vi "HFRR ADV v039.vi"() -> ()   [LabVIEW 2025] (continued)
            n794 = local write "Friction Force Tab"(T25."Page 1" ("Friction Force Tab")) -> ()
            n795 = local write "Main Calibration Tab"(T7."Main" ("Main Calibration Tab")) -> ()
          }
        }
      }
      event "FF CONTINUE": Value Change {
        n796 = event-data() -> ()  [unwired: 1 in, 6 out]
        n797 = local write "FF CONTINUE"(FALSE ("FF CONTINUE")) -> ()
        n798 = local write "Friction Force Tab"(T25."Page 2" ("Friction Force Tab")) -> ()
      }
      event "FF CONTINUE 2": Value Change {
        n799 = event-data() -> ()  [unwired: 1 in, 6 out]
        n800 = local write "FF CONTINUE 2"(FALSE ("FF CONTINUE")) -> ()
        n801 = local write "Friction Force Tab"(T25."Page 3" ("Friction Force Tab")) -> ()
      }
      event "FF CONTINUE 3": Value Change {
        n802 = event-data() -> ()  [unwired: 1 in, 6 out]
        n803 = local write "FF CONTINUE 3"(FALSE ("FF CONTINUE")) -> ()
        n804 = local write "Friction Force Tab"(T25."Page 4" ("Friction Force Tab")) -> ()
      }
      event "FF CONTINUE 4": Value Change {
        n805 = event-data() -> ()  [unwired: 1 in, 6 out]
        n806 = local write "FF CONTINUE 4"(FALSE ("FF CONTINUE")) -> ()
        n807 = local write "Friction Force Tab"(T25."Page 5" ("Friction Force Tab")) -> ()
      }
      event "FF CONTINUE 5": Value Change {
        n808 = event-data() -> ()  [unwired: 1 in, 6 out]
        n809 = local write "FF CONTINUE 5"(FALSE ("FF CONTINUE")) -> ()
        n810 = local write "Friction Force Tab"(T25."Page 6" ("Friction Force Tab")) -> ()
      }
      event "Quit": Value Change {
        n811 = event-data() -> ()  [unwired: 1 in, 6 out]
      }
    }
    n812 = Wait (ms)(milliseconds to wait=u32 100) -> ()  [unwired: 1 out]
  }
  n813 = while {
    shift-right: [w834] -> _
    shift-left: "Enum - Selector" -> [w835]
    stop <- w836 stop-if-true
    # "Auto Start Logic Loop"
    n814 = case shown="\"close\"" w835 {
      tunnel: [w839 w845 w872 w904 w934 Auto_Start_enum."Exit" ("Enum - Selector") Auto_Start_enum."Init" ("Enum - Selector")] -> w834
      frame "Init", Default {
        n815 = local read "Auto Start Test"() -> (w838:bool)
        n816 = Select(t=Auto_Start_enum."Humidity & Temperature On" ("Enum - Selector"), s=w838, f=Auto_Start_enum."Init") -> (s? t:f=w839:T15)
      }
      frame "Humidity & Temperature On" {
        n817 = stacked-sequence {
          tunnel: [_ _ _ _ _ _ Auto_Start_enum."Reach point" ("Enum - Selector")] -> w842
          frame #0 {
            w847 = T19."Disabled and Grayed Out" ("Disabled")
            w848 = TRUE ("Heater Button")
            n818 = property on="Humidity" class="Bool (strict)"("DisabledEnum"=w847) -> ()  [unwired: 2 in, 2 out]
            n819 = property on="Heater Button" class="Bool (strict)"("DisabledEnum"=w847) -> ()  [unwired: 2 in, 2 out]
            n820 = local write "Heater Button"(w848) -> ()
            n821 = local write "Humidity"(w848) -> ()
            n822 = property on="Heater Button" class="Bool (strict)"("Val(Sgnl)"=TRUE ("Value (Signaling)")) -> ()  [unwired: 2 in, 2 out]
          }
          frame #1 {
            n823 = Wait (ms)(milliseconds to wait=u32 3000) -> ()  [unwired: 1 out]
          }
          frame #2 {
            n824 = local read "Set Temp"() -> (w854:dbl)
            n825 = Number To Fractional String(number=w854, precision (6)=i16 2) -> (F-format string=w851:string)  [unwired: 2 in]
            n826 = Concatenate Strings("ST;" ("Command"), w851) -> (w852:string)
            n827 = local write "Due Write"(w852) -> ()
          }
          frame #3 {
            n828 = Wait (ms)(milliseconds to wait=u32 1500) -> ()  [unwired: 1 out]
          }
          frame #4 {
            (unwired) i16 2 ("precision (6)")
            n829 = local read "WriteHumidity"() -> (w856:string[])
            n830 = local read "Set Rh"() -> (w859:dbl)
            n831 = Number To Fractional String(number=w859) -> (F-format string=w860:string)  [unwired: 3 in]
            n832 = Concatenate Strings("M;" ("new element/subarray"), w860) -> (w861:string)
            n833 = Insert Into Array(array=w856, new element=w861) -> (w857:string[])  [unwired: 1 in]
            n834 = local write "WriteHumidity"(w857) -> ()
            n835 = local write "Due Write"("HE;1" ("Command")) -> ()
          }
          frame #5 {
            n836 = Wait (ms)(milliseconds to wait=u32 1500) -> ()  [unwired: 1 out]
          }
          frame #6 {
            w864 = TRUE ("Reach point temp")
            n837 = local write "Reach point Humidity"(w864) -> ()
            n838 = local write "Reach point temp"(w864) -> ()
          }
        }
        n839 = local read "Auto Start Test"() -> (w844:bool)
        n840 = Not(x=w844) -> (.not. x?=w843:bool)
        n841 = Select(t=Auto_Start_enum."close", s=w843, f=w842) -> (s? t:f=w845:T15)
      }
      frame "Reach point" {
        w873 = TRUE ("PAUSE")
        w881 = 1.0 ("y")
        w884 = 1.0 ("y")
        n842 = local read "Set Temp"() -> (w866:dbl)
        n843 = local read "Set Humidity:"() -> (w880:dbl)
        n844 = local read "Humidity ( %RH )"() -> (w885:dbl)
        n845 = Add(x=w866, y=w884) -> (x+y=w883:dbl)
        n846 = Subtract(x=w866, y=w884) -> (x-y=w882:dbl)
        n847 = Add(x=w880, y=w881) -> (x+y=w879:dbl)
        n848 = Subtract(x=w880, y=w881) -> (x-y=w878:dbl)
        n849 = local read "TEMP"() -> (w886:dbl)
        n850 = In Range and Coerce(upper limit=w879, x=w885, lower limit=w878) -> (In Range?=w867:bool)  [unwired: 1 out]
        n851 = In Range and Coerce(upper limit=w883, x=w886, lower limit=w882) -> (In Range?=w868:bool)  [unwired: 1 out]
        n852 = case shown="True" w867 {
          frame False {
          }
          frame True {
            n853 = case shown="True" "Reach point Humidity" {
              selector: "Reach point Humidity" -> [_ w892]
              frame False {
              }
              frame True {
                n854 = local read "EVENT LOG"() -> (w889:string)
                n855 = Not(x=w892) -> (.not. x?=w891:bool)
                n856 = local write "Reach point Humidity"(w891) -> ()
                n857 = call "Event Log.vi"("Content"="Target Humidity reached", "EVENT LOG"=w889) -> ("EVENT LOG"=w890:string)  [unwired: 8 in, 1 out]
                n858 = local write "EVENT LOG"(w890) -> ()
              }
            }
          }
        }
        n859 = case shown="True" w868 {
          frame False {
          }
          frame True {
            n860 = case shown="True" "Reach point temp" {
              selector: "Reach point temp" -> [_ w898]
              frame False {
              }
              frame True {
                n861 = local read "EVENT LOG"() -> (w895:string)
                n862 = Not(x=w898) -> (.not. x?=w897:bool)
                n863 = local write "Reach point temp"(w897) -> ()
                n864 = call "Event Log.vi"("Content"="Target Temperature reached", "EVENT LOG"=w895) -> ("EVENT LOG"=w896:string)  [unwired: 8 in, 1 out]
                n865 = local write "EVENT LOG"(w896) -> ()
              }
            }
          }
        }
        n866 = local read "Auto Start Test"() -> (w871:bool)
        n867 = And(x=w868, y=w867) -> (x .and. y?=w877:bool)
        n868 = Select(t=Auto_Start_enum."Maintain Stage" ("Enum - Selector"), s=w877, f=Auto_Start_enum."Reach point" ("Enum - Selector")) -> (s? t:f=w874:T15)
        n869 = Not(x=w871) -> (.not. x?=w870:bool)
        n870 = Select(t=Auto_Start_enum."close", s=w870, f=w874) -> (s? t:f=w872:T15)
        n871 = call "ELAPSED TIMER VI.vi"("RESET"=w873, "PAUSE"=w873) -> ()  [unwired: 7 in, 3 out]
      }
      frame "Maintain Stage" {
        w913 = 2.0 ("y")
        w912 = 1.0 ("y")
        # "Humidity and  temperatures Set Point  have been reached"
        n872 = local read "Set Temp"() -> (w899:dbl)
        n873 = local read "Set Humidity:"() -> (w916:dbl)
        n874 = local read "Humidity ( %RH )"() -> (w919:dbl)
        n875 = Add(x=w899, y=w912) -> (x+y=w918:dbl)
        n876 = Subtract(x=w899, y=w912) -> (x-y=w917:dbl)
        n877 = local read "TEMP"() -> (w920:dbl)
        n878 = Add(x=w916, y=w913) -> (x+y=w915:dbl)
        n879 = Subtract(x=w916, y=w913) -> (x-y=w914:dbl)
        n880 = In Range and Coerce(upper limit=w918, x=w920, lower limit=w917) -> (In Range?=w911:bool)  [unwired: 1 out]
        n881 = In Range and Coerce(upper limit=w915, x=w919, lower limit=w914) -> (In Range?=w910:bool)  [unwired: 1 out]
        n882 = And(x=w911, y=w910) -> (x .and. y?=w909:bool)
        n883 = Not(x=w909) -> (.not. x?=w908:bool)
        n884 = call "ELAPSED TIMER VI.vi"("TARGET"=60.0, "RESET"=w908, "PAUSE"=FALSE) -> ("ELAPSED INDICATION"=w905:bool)  [unwired: 6 in, 2 out]
        n885 = case shown="True" w905 {
          tunnel: w905 -> [_ w923]
          tunnel: [Auto_Start_enum."Maintain Stage" ("Enum - Selector") w922] -> w903
          frame False {
          }
          frame True {
            n886 = stacked-sequence {
              tunnel: w923 -> [_ _ _ _ _]
              tunnel: [_ _ _ _ Auto_Start_enum."Start Stage" ("Enum - Selector")] -> w922
              frame #0 {
                n887 = local read "EVENT LOG"() -> (w925:string)
                n888 = call "Event Log.vi"("Content"="Humidity and temperature set point has stabilized.", "EVENT LOG"=w925) -> ("EVENT LOG"=w926:string)  [unwired: 8 in, 1 out]
                n889 = local write "EVENT LOG"(w926) -> ()
              }
              frame #1 {
                n890 = Wait (ms)(milliseconds to wait=u32 100) -> ()  [unwired: 1 out]
              }
              frame #2 {
                n891 = local read "EVENT LOG"() -> (w929:string)
                n892 = call "Event Log.vi"("Content"="Auto Test Started", "EVENT LOG"=w929) -> ("EVENT LOG"=w930:string)  [unwired: 8 in, 1 out]
                n893 = local write "EVENT LOG"(w930) -> ()
              }
              frame #3 {
                w931 = TRUE ("RUN")
                n894 = local write "RUN"(w931) -> ()
                n895 = property on="Auto Start Temp" class="Bool (strict)"("Val(Sgnl)"=w931) -> ()  [unwired: 2 in, 2 out]
                "Auto Start Temp" <- w931
              }
              frame #4 {
              }
            }
          }
        }
        n896 = local read "Auto Start Test"() -> (w902:bool)
        n897 = Not(x=w902) -> (.not. x?=w901:bool)
        n898 = Select(t=Auto_Start_enum."close", s=w901, f=w903) -> (s? t:f=w904:T15)
      }
      frame "Start Stage" {
        w933 = TRUE ("PAUSE")
        n899 = local read "Auto Start Test"() -> (w938:bool)
        n900 = Not(x=w938) -> (.not. x?=w937:bool)
        n901 = Select(t=Auto_Start_enum."close" ("Enum - Selector"), s=w937, f=Auto_Start_enum."Start Stage" ("Enum - Selector")) -> (s? t:f=w934:T15)
        n902 = call "ELAPSED TIMER VI.vi"("RESET"=w933, "PAUSE"=w933) -> ()  [unwired: 7 in, 3 out]
      }
      frame "close" {
        w941 = FALSE ("Heater Button")
        n903 = local write "RUN"(w941) -> ()
        n904 = local write "Heater Button"(w941) -> ()
        n905 = local write "Humidity"(w941) -> ()
        n906 = local write "Auto Start Test"(w941) -> ()
        n907 = property on="Heater Button" class="Bool (strict)"("Val(Sgnl)"=FALSE ("Value (Signaling)")) -> ()  [unwired: 2 in, 2 out]
        n908 = local write "Humidity 2"(TRUE ("Humidity")) -> ()
      }
      frame "Exit" {
      }
    }
    n909 = Wait (ms)(milliseconds to wait=u32 100) -> ()  [unwired: 1 out]
    n910 = local read "Quit"() -> (w836:bool)
  }
  n911 = property on="Service Password Log" class="Str"("Visible"=w21) -> ()  [unwired: 2 in, 2 out]
  n912 = property on="Password 3" class="Clust (strict)"("Visible"=w21) -> ()  [unwired: 2 in, 2 out]
  n913 = while {
    stop <- w970 stop-if-true
    w953 = errorcluster {"status"=FALSE, "code"=0, "source"=""} ("error in (no error) 3")
    # "this loop is for manual report generation"
    n914 = local read "Confirm Measrurement"() -> (w952:bool)
    n915 = case shown="True" w952 {
      selector: w952 -> [_ w1060]
      tunnel: errorcluster {"status"=FALSE, "code"=0, "source"=""} ("error in (no error) 3") -> [_ w1061]
      tunnel: [_ w1059] -> _
      frame False {
      }
      frame True {
        n916 = stacked-sequence {
          tunnel: w1061 -> [_ w1094 _]
          tunnel: w1060 -> [_ _ w1201]
          tunnel: [_ w1082 _] -> w1059
          frame #0 {
            n917 = String To Path(string="C:\\LAB-IQ\\Image Calibrate v01.dcf") -> (path=w1064:path)
            n918 = Open/Create/Replace File ("Open File")(file path (use dialog)=w1064) -> (refnum out=w1065:refnum<file>)  [unwired: 5 in, 2 out]
            n919 = for {
              N: 4 -> [_]
              tunnel: w1065 -> [w1071]
              i -> [w1067]
              n920 = Read from Text File ("Read File")(file (use dialog)=w1071) -> (text=w1072:string)  [unwired: 3 in, 3 out]
              n921 = String Subset(string=w1072, offset (0)=6, length (rest)=10 ("length (rest)")) -> (substring=w1068:string)
              n922 = Fract/Exp String To Number(string=w1068) -> (number=w1066:dbl)  [unwired: 3 in, 1 out]
              n923 = case shown="3" w1067 {
                tunnel: w1066 -> [w1073 w1074 _ w1075 _]
                frame 0 {
                  n924 = local write "5x Gain"(w1073) -> ()
                }
                frame 1 {
                  n925 = local write "10x Gain"(w1074) -> ()
                }
                frame 2 {
                }
                frame 3 {
                  n926 = local write "100x gain"(w1075) -> ()
                }
                frame 4, Default {
                }
              }
            }
          }
          frame #1 {
            n927 = local read "TEST STANDARD"() -> (w1077:T3)
            n928 = case shown="\"ISO 12156\"" w1077 {
              tunnel: ["ASTM D6079" "ISO 12156"] -> w1076
              frame "ASTM D6079", Default {
              }
              frame "ISO 12156" {
              }
            }
            n929 = call "IMAGE ANALYSIS.vi"("Enum"=POST_ANALYSIS_ENUM."GET MEASUREMENTS", "error in"=w1094) -> ("error out"=w1101:errorcluster)  [unwired: 8 in, 1 out]
            n930 = local read "Magnification :"() -> (w1087:string)
            n931 = call "Stall Data Flow.vim"("value in"=w1101, "milliseconds to wait"=u32 1000) -> ("value out"=w1100:errorcluster)  [unwired: 1 out]
            n932 = local read "Test File List :"() -> (w1098:string)
            n933 = case shown="\"10x\"" w1087 {
              tunnel: [w1137 w1138] -> w1085
              frame "5x", Default {
                n934 = local read "5x Gain"() -> (w1137:dbl)
              }
              frame "10x" {
                # "5x"
                n935 = local read "10x Gain"() -> (w1138:dbl)
              }
            }
            n936 = call "IMAGE ANALYSIS.vi"("Enum"=POST_ANALYSIS_ENUM."READ", "error in"=w1100) -> ("error out"=w1097:errorcluster, "data out"=w1088:string)  [unwired: 8 in]
            n937 = Match Pattern(string=w1088, regular expression="\"type\": ") -> (after substring=w1092:string)  [unwired: 1 in, 3 out]
            n938 = call "IMAGE PATH CREATION PY.vi"("error in (no error)"=w1097, "File Name :"=w1098) -> ("error out"=w1096:errorcluster, "File Path"=w1084:path, "File Path String:"=w1079:string)  [unwired: 7 in]
            n939 = Match Pattern(string=w1092, regular expression=",") -> (before substring=w1078:string)  [unwired: 1 in, 3 out]
            n940 = local read "Calibration Tab"() -> (w1081:enum32{"Measrument", "Calibrate"})
            n941 = call "Stall Data Flow.vim"("value in"=w1096, "milliseconds to wait"=u32 250) -> ("value out"=w1080:errorcluster)  [unwired: 1 out]
            n942 = Equal?(x=w1078, y="\"rectangle\"") -> (x = y?=w1089:bool)
            n943 = case shown="False" w1089 {
              tunnel: w1088 -> [w1143 w1198]
              tunnel: w1085 -> [_ w1189]
              tunnel: cluster{"major":dbl, "minor":dbl, "average":dbl} {"major"=0.0, "minor"=0.0, "average"=0.0} -> [w1141 w1185]
              tunnel: [w1140 w1182] -> w1083
              tunnel: w1078 -> [w1142 _]
              tunnel: w1085 -> [w1139 _]
              frame False {
                n944 = Equal?(x=w1142, y="\"line\"") -> (x = y?=w1144:bool)
                n945 = case shown="True" w1144 {
                  tunnel: w1143 -> [_ w1159]
                  tunnel: w1141 -> [w1146 w1158]
                  tunnel: [w1146 w1156] -> w1140
                  tunnel: w1139 -> [_ w1155]
                  frame False {
                  }
                  frame True {
                    w1154 = 0.0 ("Major Axis")
                    n946 = Match Pattern(string=w1159, regular expression="\"length_px\":") -> (after substring=w1157:string)  [unwired: 1 in, 3 out]
                    n947 = property on="Major Axis" class="DigNum (strict)"("Caption.Text"="") -> ()  [unwired: 2 in, 2 out]
                    n948 = property on="Minor Axis" class="DigNum (strict)"("Caption.Text"="") -> ()  [unwired: 2 in, 2 out]
                    n949 = property on="Average" class="DigNum (strict)"("Caption.Text"="Line") -> ()  [unwired: 2 in, 2 out]
                    n950 = Fract/Exp String To Number(string=w1157, default (0 dbl)=0.0 ("default (0 DBL)")) -> (number=w1153:dbl)  [unwired: 2 in, 1 out]
                    "Pixel Value" <- w1153
                    n951 = Multiply(x=w1153, y=w1155) -> (x*y=w1166:dbl)
                    n952 = Multiply(x=w1166, y=1000.0) -> (x*y=w1149:dbl)
                    n953 = Divide(x=w1149, y=1000.0) -> (x/y=w1152:dbl)
                    n954 = local write "Measurment (mm)"(w1152) -> ()
                    n955 = Bundle By Name(cluster=w1158, "average"=w1149) -> (w1156:cluster{"major":dbl, "minor":dbl, "average":dbl})
                    n956 = Number To Fractional String(number=w1149, precision (6)=i16 1) -> (F-format string=w1148:string)  [unwired: 2 in]
                    n957 = local write "Minor Axis"(w1154) -> ()
                    n958 = local write "Major Axis"(w1154) -> ()
                    n959 = Fract/Exp String To Number(string=w1148) -> (number=w1147:dbl)  [unwired: 3 in, 1 out]
                    n960 = local write "Average"(w1147) -> ()
                  }
                }
              }
              frame True {
                w1186 = 1000.0 ("y")
                w1192 = 0.0 ("default (0 DBL)")
                n961 = Match Pattern(string=w1198, regular expression=" \"width_px\":") -> (after substring=w1196:string)  [unwired: 1 in, 3 out]
                n962 = Match Pattern(string=w1196, regular expression="\"height_px\":") -> (before substring=w1194:string, after substring=w1193:string)  [unwired: 1 in, 2 out]
                n963 = Fract/Exp String To Number(string=w1194, default (0 dbl)=w1192) -> (number=w1191:dbl)  [unwired: 2 in, 1 out]
                n964 = Fract/Exp String To Number(string=w1193, default (0 dbl)=w1192) -> (number=w1190:dbl)  [unwired: 2 in, 1 out]
                n965 = Multiply(x=w1191, y=w1189) -> (x*y=w1188:dbl)
                n966 = Multiply(x=w1190, y=w1189) -> (x*y=w1187:dbl)
                n967 = Multiply(x=w1188, y=w1186) -> (x*y=w1172:dbl)
                n968 = Multiply(x=w1187, y=w1186) -> (x*y=w1170:dbl)
                n969 = Add(x=w1172, y=w1170) -> (x+y=w1184:dbl)
                n970 = property on="Major Axis" class="DigNum (strict)"("Caption.Text"="Major Axis") -> ()  [unwired: 2 in, 2 out]
                n971 = property on="Minor Axis" class="DigNum (strict)"("Caption.Text"="Minor Axis") -> ()  [unwired: 2 in, 2 out]
                n972 = property on="Average" class="DigNum (strict)"("Caption.Text"="Average") -> ()  [unwired: 2 in, 2 out]
                n973 = Divide(x=w1184, y=2.0) -> (x/y=w1168:dbl)
                n974 = Bundle By Name(cluster=w1185, "major"=w1172, "minor"=w1170, "average"=w1168) -> (w1182:cluster{"major":dbl, "minor":dbl, "average":dbl})
                n975 = Number To Fractional String(number=w1170, precision (6)=i16 1) -> (F-format string=w1177:string)  [unwired: 2 in]
                n976 = Number To Fractional String(number=w1168, precision (6)=i16 1) -> (F-format string=w1178:string)  [unwired: 2 in]
                n977 = Number To Fractional String(number=w1172, precision (6)=i16 1) -> (F-format string=w1176:string)  [unwired: 2 in]
                n978 = Fract/Exp String To Number(string=w1177) -> (number=w1169:dbl)  [unwired: 3 in, 1 out]
                n979 = Fract/Exp String To Number(string=w1178) -> (number=w1167:dbl)  [unwired: 3 in, 1 out]
                n980 = Fract/Exp String To Number(string=w1176) -> (number=w1171:dbl)  [unwired: 3 in, 1 out]
                n981 = local write "Major Axis"(w1171) -> ()
                n982 = local write "Average"(w1167) -> ()
                n983 = local write "Minor Axis"(w1169) -> ()
              }
            }
            n984 = case shown="\"Measrument\", Default" w1081 {
              tunnel: w1084 -> [w1111 _]
              tunnel: w1083 -> [w1110 _]
              tunnel: [w1107 w1136] -> w1082
              tunnel: w1080 -> [w1109 w1136]
              tunnel: w1079 -> [w1108 _]
              tunnel: w1076 -> [w1106 _]
              frame "Measrument", Default {
                n985 = stacked-sequence {
                  tunnel: w1111 -> [w1129 _]
                  tunnel: w1110 -> [w1127 _]
                  tunnel: w1109 -> [w1125 _]
                  tunnel: w1108 -> [w1124 _]
                  tunnel: [w1119 _] -> w1107
                  tunnel: w1106 -> [w1112 _]
                  frame #0 {
                    n986 = call "IMAGE ANALYSIS.vi"("Enum"=POST_ANALYSIS_ENUM."SAVE IMAGE", "error in"=w1125, "IMAGE FILE PATH"=w1124) -> ("error out"=w1123:errorcluster)  [unwired: 7 in, 1 out]
                    n987 = call "Stall Data Flow.vim"("value in"=w1123, "milliseconds to wait"=u32 1000) -> ("value out"=w1114:errorcluster)  [unwired: 1 out]
                    n988 = local read "Test File List :"() -> (w1131:string)
                    n989 = call "IMAGE ANALYSIS.vi"("Enum"=POST_ANALYSIS_ENUM."MINIMIZE UI", "error in"=w1114) -> ("error out"=w1121:errorcluster)  [unwired: 8 in, 1 out]
                    n990 = Bundle By Name(cluster=T27 {"File Name"="", "Test Method"="", "Operator"="", "Fuel Description"="", "Date and time"=""} ("Main Ref"), "Test Method"=w1112, "File Name"=w1131) -> (w1132:T27)
                    n991 = call "Stall Data Flow.vim"("value in"=w1121, "milliseconds to wait"=u32 1500) -> ("value out"=w1116:errorcluster)  [unwired: 1 out]
                    n992 = call "duf file read.vi"("error in (no error)"=w1116, "Main Ref"=w1132) -> ("error out"=w1130:errorcluster, "Main Ref 2"=w1128:T27)  [unwired: 8 in]
                    n993 = call "DETECTION REPORT for manual.vi"("error in (no error)"=w1130, "return value 3"=w1127, "Image File Path"=w1129, "Main Ref"=w1128) -> ("error out"=w1126:errorcluster)  [unwired: 7 in]
                    n994 = call <vilib>:"Clear Errors.vi"("error in (no error)"=w1126) -> ("error out"=w1117:errorcluster)  [unwired: 5 in, 1 out]
                    n995 = call "IMAGE ANALYSIS.vi"("Enum"=POST_ANALYSIS_ENUM."MINIMIZE UI", "error in"=w1117) -> ("error out"=w1119:errorcluster)  [unwired: 8 in, 1 out]
                  }
                  frame #1 {
                    n996 = local write "Main Tab"(T2."HOME" ("Main Tab")) -> ()
                    n997 = local write "Main Dashboard Buttons"(T1."Home" ("Main Dashboard Buttons")) -> ()
                  }
                }
              }
              frame "Calibrate" {
              }
            }
          }
          frame #2 {
            n998 = Not(x=w1201) -> (.not. x?=w1200:bool)
            n999 = local write "Confirm Measrurement"(w1200) -> ()
            n1000 = local read "Calibration Tab"() -> (w1199:enum32{"Measrument", "Calibrate"})
            n1001 = case shown="\"Measrument\", Default" w1199 {
              frame "Measrument", Default {
                (unwired) T21."HOME" ("Main Tab")
                n1002 = local write "Main Tab"(T2."HOME" ("Main Tab")) -> ()
              }
              frame "Calibrate" {
              }
            }
          }
        }
      }
    }
    n1003 = local read "Humidity"() -> (w944:bool)
    n1004 = local read "Save Change"() -> (w949:bool)
    n1005 = local read "Calibrate"() -> (w950:bool)
    n1006 = local read "Auto Start Test"() -> (w945:bool)
    n1007 = case shown="True" w950 {
      selector: w950 -> [_ w1057]
      frame False {
      }
      frame True {
        n1008 = Not(x=w1057) -> (.not. x?=w1056:bool)
        n1009 = local write "Calibrate"(w1056) -> ()
        n1010 = local write "Calibration Tab"(enum32{"Measrument", "Calibrate"}."Calibrate" ("Calibration Tab")) -> ()
      }
    }
    n1011 = case shown="True" w949 {
      selector: w949 -> [_ w1001]
      frame False {
      }
      frame True {
        n1012 = stacked-sequence {
          tunnel: w1001 -> [_ _ _ _ w1055]
          frame #0 {
            n1013 = call "IMAGE ANALYSIS.vi"("Enum"=POST_ANALYSIS_ENUM."HIDE UI") -> ()  [unwired: 9 in, 2 out]
          }
          frame #1 {
            n1014 = local read "100x gain"() -> (w1003:dbl)
            n1015 = local read "10x Gain"() -> (w1004:dbl)
            n1016 = local read "5x Gain"() -> (w1005:dbl)
            n1017 = Number To Fractional String(number=w1004, width (-)=i16 4, precision (6)=i16 7) -> (F-format string=w1026:string)  [unwired: 1 in]
            n1018 = Number To Fractional String(number=0.0, width (-)=i16 4, precision (6)=i16 7) -> (F-format string=w1021:string)  [unwired: 1 in]
            n1019 = Number To Fractional String(number=w1003, width (-)=i16 4, precision (6)=i16 7) -> (F-format string=w1009:string)  [unwired: 1 in]
            n1020 = Number To Fractional String(number=w1005, width (-)=i16 10 ("precision (6)"), precision (6)=i16 7) -> (F-format string=w1035:string)  [unwired: 1 in]
            n1021 = Concatenate Strings("[CH1]" ("string"), w1035, " - 5x Gain" ("string"), "\r") -> (w1025:string)
            n1022 = Concatenate Strings("[CH2]" ("string"), w1026, " - 10x Gain" ("string"), "\r") -> (w1024:string)
            n1023 = Concatenate Strings("[CH3]" ("string"), w1021, " - 20x Gain" ("string"), "\r") -> (w1015:string)
            n1024 = Concatenate Strings("[CH4]" ("string"), w1009, " - 100x Gain" ("string"), "\r") -> (w1008:string)
            n1025 = String To Path(string="C:\\LAB-IQ\\Image Calibrate v01.dcf") -> (path=w1038:path)
            n1026 = Concatenate Strings(w1025, w1024, w1015, w1008) -> (w1023:string)
            n1027 = call <vilib>:"Write Characters To File.vi"("append to file? (new file:F)"=FALSE, "character string"=w1023, "file path (dialog if empty)"=w1038) -> ()  [unwired: 2 in, 1 out]
          }
          frame #2 {
            n1028 = String To Path(string="C:\\LAB-IQ\\Image Calibrate v01.dcf") -> (path=w1041:path)
            n1029 = Open/Create/Replace File ("Open File")(file path (use dialog)=w1041) -> (refnum out=w1042:refnum<file>)  [unwired: 5 in, 2 out]
            n1030 = for {
              N: 4 -> [_]
              tunnel: w1042 -> [w1048]
              i -> [w1044]
              n1031 = Read from Text File ("Read File")(file (use dialog)=w1048) -> (text=w1049:string)  [unwired: 3 in, 3 out]
              n1032 = String Subset(string=w1049, offset (0)=6, length (rest)=10 ("length (rest)")) -> (substring=w1045:string)
              n1033 = Fract/Exp String To Number(string=w1045) -> (number=w1043:dbl)  [unwired: 3 in, 1 out]
              n1034 = case shown="3" w1044 {
                tunnel: w1043 -> [w1050 w1051 _ w1052 _]
                frame 0 {
                  n1035 = local write "5x Gain"(w1050) -> ()
                }
                frame 1 {
                  n1036 = local write "10x Gain"(w1051) -> ()
                }
                frame 2 {
                }
                frame 3 {
                  n1037 = local write "100x gain"(w1052) -> ()
                }
                frame 4, Default {
                }
              }
            }
          }
          frame #3 {
            n1038 = call "IMAGE ANALYSIS.vi"("Enum"=POST_ANALYSIS_ENUM."SHOW UI") -> ()  [unwired: 9 in, 2 out]
          }
          frame #4 {
            n1039 = Not(x=w1055) -> (.not. x?=w1054:bool)
            n1040 = local write "Save Change"(w1054) -> ()
          }
        }
      }
    }
    n1041 = case shown="False" w945 {
      tunnel: w944 -> [w971 _]
      frame False {
        n1042 = case shown="True" w971 {
          frame False {
          }
          frame True {
            n1043 = local read "Set Humidity:"() -> (w975:dbl)
            n1044 = local read "Set Humidity:"() -> (w978:dbl)
            n1045 = local read "Humidity ( %RH )"() -> (w979:dbl)
            n1046 = Subtract(x=w975, y=2.0) -> (x-y=w973:dbl)
            n1047 = Add(x=w978, y=2.0) -> (x+y=w974:dbl)
            n1048 = In Range and Coerce(upper limit=w974, x=w979, lower limit=w973) -> (In Range?=w972:bool)  [unwired: 1 out]
            n1049 = case shown="True" w972 {
              frame False {
              }
              frame True {
                n1050 = case shown="True" "Manual Humididty Reached" {
                  selector: "Manual Humididty Reached" -> [_ w982]
                  frame False {
                  }
                  frame True {
                    n1051 = Not(x=w982) -> (.not. x?=w981:bool)
                    n1052 = local write "Manual Humididty Reached"(w981) -> ()
                    n1053 = local read "EVENT LOG"() -> (w984:string)
                    n1054 = call "Event Log.vi"("Content"="Target Humidity reached", "EVENT LOG"=w984) -> ("EVENT LOG"=w983:string)  [unwired: 8 in, 1 out]
                    n1055 = local write "EVENT LOG"(w983) -> ()
                  }
                }
              }
            }
          }
        }
      }
      frame True {
        n1056 = local write "Manual Humididty Reached"(TRUE ("Manual Humididty Reached")) -> ()
      }
    }
    n1057 = local read "Cap Live Image"() -> (w965:bool)
    n1058 = local read "SCAR MEASURMENT"() -> (w968:enum32{"Auto Scar", "Manual Scar"})
    n1059 = Equal?(x=w968, y=enum32{"Auto Scar", "Manual Scar"}."Manual Scar" ("SCAR MEASURMENT")) -> (x = y?=w966:bool)
    n1060 = And(x=w966, y=w965) -> (x .and. y?=w964:bool)
    n1061 = Wait (ms)(milliseconds to wait=u32 250) -> ()  [unwired: 1 out]
    n1062 = case shown="True" w964 {
      selector: w964 -> [_ w1287]
      frame False {
      }
      frame True {
        n1063 = stacked-sequence {
          tunnel: [_ _ _ w1306 _] -> _
          tunnel: w1287 -> [_ _ _ _ w1313]
          frame #0 {
            w1288 = 0.0
            n1064 = local write "Major Axis"(w1288) -> ()
            n1065 = local write "Minor Axis"(w1288) -> ()
            n1066 = local write "Average"(w1288) -> ()
          }
          frame #1 {
            n1067 = call "CAMERA LIVE FEED FGV.vi"("Enum - Menu"=CAMERA_LIVE_FEED_ENUM."CAMERA MINIMIZE") -> ()  [unwired: 9 in, 2 out]
          }
          frame #2 {
            n1068 = local read "Magnification len live scar"() -> (w1292:string)
            n1069 = case shown="\"10x\", Default" w1292 {
              tunnel: ["_10x" "_5x"] -> w1291
              frame "10x", Default {
              }
              frame "5x" {
              }
            }
            n1070 = local read "FILE 3"() -> (w1298:string)
            n1071 = call <vilib>:"Trim Whitespace.vi"("string"="C:\\LAB-IQ\\images\\") -> ("trimmed string"=w1300:string)  [unwired: 1 in]
            n1072 = String To Path(string=w1300) -> (path=w1299:path)
            n1073 = Concatenate Strings(w1298, w1291, ".png" ("string")) -> (w1297:string)
            n1074 = Build Path(base path=w1299, name or relative path=w1297) -> (appended path=w1296:path)
            n1075 = Path To String(path=w1296) -> (string=w1295:string)
            n1076 = call "CAMERA LIVE FEED FGV.vi"("Enum - Menu"=CAMERA_LIVE_FEED_ENUM."CAMERA SAVE", "Image Path"=w1295) -> ("error out"=w1293:errorcluster)  [unwired: 8 in, 1 out]
            n1077 = case shown="No Error" w1293 {
              frame No Error {
                n1078 = One Button Dialog(message="Image saved successfully") -> ()  [unwired: 1 in, 1 out]
              }
              frame Error {
              }
            }
          }
          frame #3 {
            n1079 = call "LIST FILE NAMES.vi"() -> ("error out"=w1308:errorcluster, "filenames"=w1305:string[])  [unwired: 10 in]
            n1080 = call "IMAGE ANALYSIS.vi"("Enum"=POST_ANALYSIS_ENUM."SHOW UI", "error in"=w1308) -> ("error out"=w1306:errorcluster)  [unwired: 8 in, 1 out]
            n1081 = property on="Test File List :" class="CmbBox"("Strings[]"=w1305) -> ()  [unwired: 2 in, 2 out]
          }
          frame #4 {
            (unwired) T26."Report" ("Main Dashboard Buttons")
            (unwired) T28."Report" ("Main Dashboard Buttons")
            n1082 = Not(x=w1313) -> (.not. x?=w1312:bool)
            n1083 = local write "Zoom Factore"(0.0 ("Zoom Factore")) -> ()
            n1084 = local write "Cap Live Image"(w1312) -> ()
            n1085 = local write "Main Tab"(T2."Adv Scar Report" ("Main Tab")) -> ()
            n1086 = property on="Cap Live Image" class="Bool (strict)"("BoolText.Text"="Capture Image" ("Boolean Text.Text")) -> ()  [unwired: 2 in, 2 out]
            n1087 = local write "Main Dashboard Buttons"(T1."Report" ("Main Dashboard Buttons")) -> ()
          }
        }
      }
    }
    n1088 = local read "change Gain"() -> (w948:bool)
    n1089 = local read "Back Square"() -> (w947:bool)
    n1090 = case shown="True" w948 {
      selector: w948 -> [_ w992]
      frame False {
      }
      frame True {
        n1091 = stacked-sequence {
          tunnel: w992 -> [_ w1000]
          frame #0 {
            n1092 = local read "Actual (µm)"() -> (w996:dbl)
            n1093 = local read "Pixel Value"() -> (w995:dbl)
            n1094 = local read "Magnification :"() -> (w994:string)
            n1095 = Divide(x=w996, y=w995) -> (x/y=w993:dbl)
            n1096 = case shown="\"10x\"" w994 {
              tunnel: w993 -> [w997 w998]
              frame "10x" {
                n1097 = local write "10x Gain"(w997) -> ()
              }
              frame "5x", Default {
                n1098 = local write "5x Gain"(w998) -> ()
              }
            }
          }
          frame #1 {
            n1099 = Not(x=w1000) -> (.not. x?=w999:bool)
            n1100 = local write "change Gain"(w999) -> ()
          }
        }
      }
    }
    n1101 = case shown="True" w947 {
      selector: w947 -> [_ w990]
      frame False {
      }
      frame True {
        n1102 = Not(x=w990) -> (.not. x?=w989:bool)
        n1103 = local write "Back Square"(w989) -> ()
        n1104 = local write "Calibration Tab"(enum32{"Measrument", "Calibrate"}."Measrument" ("Calibration Tab")) -> ()
      }
    }
    n1105 = local read "Rectangle Tool"() -> (w959:bool)
    n1106 = local read "Clear ROI Tool"() -> (w958:bool)
    n1107 = local read "Open Image"() -> (w963:bool)
    n1108 = local read "line tool"() -> (w960:bool)
    n1109 = local read "OUT"() -> (w961:bool)
    n1110 = local read "In"() -> (w962:bool)
    n1111 = case shown="True" w963 {
      selector: w963 -> [_ w1273]
      tunnel: [w1264 w1275] -> _
      tunnel: w953 -> [w1264 w1274]
      frame False {
      }
      frame True {
        w1268 = "_5x" ("regular expression")
        n1112 = Not(x=w1273) -> (.not. x?=w1272:bool)
        n1113 = local write "Open Image"(w1272) -> ()
        n1114 = call "IMAGE ANALYSIS.vi"("Enum"=POST_ANALYSIS_ENUM."HIDE UI", "error in"=w1274) -> ("error out"=w1282:errorcluster)  [unwired: 8 in, 1 out]
        n1115 = call <vilib>:"Clear Errors.vi"("error in (no error)"=w1282) -> ("error out"=w1265:errorcluster)  [unwired: 5 in, 1 out]
        n1116 = call "File Dialog"("start path"=path "C:/LAB-IQ/images", "error in"=w1265) -> ("selected path"=w1267:path, "error out"=w1280:errorcluster)  [unwired: 10 in, 2 out]
        "Image path  2" <- w1267
        n1117 = call <vilib>:"Clear Errors.vi"("error in (no error)"=w1280) -> ("error out"=w1279:errorcluster)  [unwired: 5 in, 1 out]
        n1118 = call "IMAGE ANALYSIS.vi"("Enum"=POST_ANALYSIS_ENUM."OPEN FILE", "error in"=w1279, "File Path"=w1267) -> ("error out"=w1278:errorcluster)  [unwired: 7 in, 1 out]
        n1119 = call <vilib>:"Clear Errors.vi"("error in (no error)"=w1278) -> ("error out"=w1277:errorcluster)  [unwired: 5 in, 1 out]
        n1120 = call "IMAGE ANALYSIS.vi"("Enum"=POST_ANALYSIS_ENUM."SHOW UI", "error in"=w1277) -> ("error out"=w1275:errorcluster)  [unwired: 8 in, 1 out]
        n1121 = local write "Zoom Factore"(100.0 ("Zoom Factore")) -> ()
        n1122 = Strip Path(path=w1267) -> (name=w1270:string)  [unwired: 1 out]
        n1123 = Match Pattern(string=w1270, regular expression=w1268) -> (match substring=w1269:string)  [unwired: 1 in, 3 out]
        n1124 = Equal?(x=w1269, y=w1268) -> (x = y?=w1266:bool)
        n1125 = case shown="False" w1266 {
          frame False {
            n1126 = local write "Magnification :"("10x" ("Magnification :")) -> ()
          }
          frame True {
            n1127 = local write "Magnification :"("5x" ("Magnification :")) -> ()
          }
        }
      }
    }
    n1128 = case shown="True" w961 {
      selector: w961 -> [_ w1249]
      tunnel: w953 -> [w1246 w1254]
      tunnel: [w1246 w1248] -> _
      frame False {
      }
      frame True {
        n1129 = Not(x=w1249) -> (.not. x?=w1247:bool)
        n1130 = local read "Zoom Factore"() -> (w1252:dbl)
        n1131 = local write "OUT"(w1247) -> ()
        n1132 = call "IMAGE ANALYSIS.vi"("Enum"=POST_ANALYSIS_ENUM."ZOOM OUT", "error in"=w1254) -> ("error out"=w1248:errorcluster)  [unwired: 8 in, 1 out]
        n1133 = Divide(x=w1252, y=1.2) -> (x/y=w1250:dbl)
        n1134 = local write "Zoom Factore"(w1250) -> ()
      }
    }
    n1135 = case shown="True" w962 {
      selector: w962 -> [_ w1258]
      tunnel: w953 -> [w1255 w1263]
      tunnel: [w1255 w1256] -> _
      frame False {
      }
      frame True {
        n1136 = Not(x=w1258) -> (.not. x?=w1257:bool)
        n1137 = local read "Zoom Factore"() -> (w1261:dbl)
        n1138 = local write "In"(w1257) -> ()
        n1139 = call "IMAGE ANALYSIS.vi"("Enum"=POST_ANALYSIS_ENUM."ZOOM IN", "error in"=w1263) -> ("error out"=w1256:errorcluster)  [unwired: 8 in, 1 out]
        n1140 = Multiply(x=w1261, y=1.2) -> (x*y=w1259:dbl)
        n1141 = local write "Zoom Factore"(w1259) -> ()
      }
    }
    n1142 = case shown="True" w958 {
      selector: w958 -> [_ w1230]
      tunnel: w953 -> [w1228 w1232]
      tunnel: [w1228 w1231] -> _
      frame False {
      }
      frame True {
        n1143 = Not(x=w1230) -> (.not. x?=w1229:bool)
        n1144 = local write "Clear ROI Tool"(w1229) -> ()
        n1145 = call "IMAGE ANALYSIS.vi"("Enum"=POST_ANALYSIS_ENUM."CLEAR ROI", "error in"=w1232) -> ("error out"=w1231:errorcluster)  [unwired: 8 in, 1 out]
      }
    }
    n1146 = case shown="True" w960 {
      selector: w960 -> [_ w1242]
      tunnel: w953 -> [w1240 w1245]
      tunnel: [w1240 w1243] -> _
      frame False {
      }
      frame True {
        n1147 = Not(x=w1242) -> (.not. x?=w1241:bool)
        n1148 = local write "line tool"(w1241) -> ()
        n1149 = call "IMAGE ANALYSIS.vi"("Enum"=POST_ANALYSIS_ENUM."DRAW LINE", "error in"=w1245) -> ("error out"=w1243:errorcluster)  [unwired: 8 in, 1 out]
      }
    }
    n1150 = case shown="True" w959 {
      selector: w959 -> [_ w1236]
      tunnel: w953 -> [w1234 w1238]
      tunnel: [w1234 w1237] -> _
      frame False {
      }
      frame True {
        n1151 = Not(x=w1236) -> (.not. x?=w1235:bool)
        n1152 = local write "Rectangle Tool"(w1235) -> ()
        n1153 = call "IMAGE ANALYSIS.vi"("Enum"=POST_ANALYSIS_ENUM."DRAW REC", "error in"=w1238) -> ("error out"=w1237:errorcluster)  [unwired: 8 in, 1 out]
      }
    }
    n1154 = local read "SCAR MEASURMENT"() -> (w946:enum32{"Auto Scar", "Manual Scar"})
    n1155 = local read "Fit to Screen Tool"() -> (w955:bool)
    n1156 = local read "Resize Tool"() -> (w954:bool)
    n1157 = case shown="\"Manual Scar\", Default" w946 {
      frame "Auto Scar" {
        n1158 = property on="Cap Live Image" class="Bool (strict)"("BoolText.Text"="Report" ("Boolean Text.Text")) -> ()  [unwired: 2 in, 2 out]
      }
      frame "Manual Scar", Default {
        n1159 = property on="Cap Live Image" class="Bool (strict)"("BoolText.Text"="Save Image" ("Boolean Text.Text")) -> ()  [unwired: 2 in, 2 out]
      }
    }
    n1160 = local read "ROI Color Tool"() -> (w956:bool)
    n1161 = local read "Pan Tool"() -> (w957:bool)
    n1162 = case shown="True" w957 {
      selector: w957 -> [_ w1224]
      tunnel: w953 -> [w1222 w1226]
      tunnel: [w1222 w1225] -> _
      frame False {
      }
      frame True {
        n1163 = Not(x=w1224) -> (.not. x?=w1223:bool)
        n1164 = call "IMAGE ANALYSIS.vi"("Enum"=POST_ANALYSIS_ENUM."PAN", "error in"=w1226) -> ("error out"=w1225:errorcluster)  [unwired: 8 in, 1 out]
        n1165 = local write "Pan Tool"(w1223) -> ()
      }
    }
    n1166 = case shown="True" w954 {
      selector: w954 -> [_ w1208]
      tunnel: w953 -> [w1203 w1205]
      tunnel: [w1203 w1204] -> _
      frame False {
      }
      frame True {
        n1167 = Not(x=w1208) -> (.not. x?=w1207:bool)
        n1168 = local write "Resize Tool"(w1207) -> ()
        n1169 = call "IMAGE ANALYSIS.vi"("Enum"=POST_ANALYSIS_ENUM."RESIZE MODE", "error in"=w1205) -> ("error out"=w1204:errorcluster)  [unwired: 8 in, 1 out]
      }
    }
    n1170 = case shown="True" w955 {
      selector: w955 -> [_ w1213]
      tunnel: [w1209 w1214] -> _
      tunnel: w953 -> [w1209 w1212]
      frame False {
      }
      frame True {
        n1171 = Not(x=w1213) -> (.not. x?=w1211:bool)
        n1172 = local write "Zoom Factore"(100.0 ("Zoom Factore")) -> ()
        n1173 = local write "Fit to Screen Tool"(w1211) -> ()
        n1174 = call "IMAGE ANALYSIS.vi"("Enum"=POST_ANALYSIS_ENUM."FIT", "error in"=w1212) -> ("error out"=w1214:errorcluster)  [unwired: 8 in, 1 out]
      }
    }
    n1175 = case shown="True" w956 {
      selector: w956 -> [_ w1219]
      tunnel: [w1216 w1220] -> _
      tunnel: w953 -> [w1216 w1217]
      frame False {
      }
      frame True {
        n1176 = Not(x=w1219) -> (.not. x?=w1218:bool)
        n1177 = local write "ROI Color Tool"(w1218) -> ()
        n1178 = call "IMAGE ANALYSIS.vi"("Enum"=POST_ANALYSIS_ENUM."SET ROI COLOR", "error in"=w1217) -> ("error out"=w1220:errorcluster)  [unwired: 8 in, 1 out]
      }
    }
    n1179 = local read "Quit"() -> (w970:bool)
  }
  n1180 = while {
    stop <- w1315 stop-if-true
    n1181 = local read "Image Path"() -> (w1318:path)
    n1182 = local read "Print 3"() -> (w1321:bool)
    n1183 = Equal?(x=w1318, y=path "") -> (x = y?=w1317:bool)
    n1184 = Not(x=w1317) -> (.not. x?=w1316:bool)
    n1185 = property on="Print 3" class="Bool (strict)"("Visible"=w1316) -> ()  [unwired: 2 in, 2 out]
    n1186 = case shown="True" w1321 {
      frame False {
        n1187 = local write "Rd"(TRUE ("Boolean 7")) -> ()
      }
      frame True {
        n1188 = flat-sequence {
          tunnel: [w1361] -> w1329
          tunnel: [w1348] -> w1327
          tunnel: [w1358] -> w1323
          tunnel: w1329 -> [w1370]
          tunnel: [w1370] -> w1328
          tunnel: w1327 -> [w1369]
          tunnel: [w1369] -> w1326
          tunnel: [w1367] -> w1325
          tunnel: [w1366] -> w1324
          tunnel: w1323 -> [w1366]
          tunnel: w1328 -> [w1372]
          tunnel: w1326 -> [w1373]
          tunnel: w1325 -> [_]
          tunnel: w1324 -> [w1371]
          frame #0 {
            n1189 = case shown="True" "Rd" {
              frame False {
              }
              frame True {
                n1190 = while {
                  tunnel: "abcdefABCDEF" ("string 2") -> [w1340]
                  shift-right: [w1338] -> w1332
                  shift-left: "" -> [w1337]
                  i -> [w1347]
                  stop <- w1346 stop-if-true
                  n1191 = Random Number (0-1)() -> (number: 0 to 1=w1341:dbl)
                  n1192 = Multiply(x=w1341, y=62.0) -> (x*y=w1343:dbl)
                  n1193 = Decrement(x="Length 2") -> (x-1=w1336:i16)
                  n1194 = To Word Integer(number=w1343) -> (16bit integer=w1344:i16)
                  n1195 = String Subset(string=w1340, offset (0)=w1344, length (rest)=1 ("length (rest)")) -> (substring=w1339:string)
                  n1196 = Greater Or Equal?(x=w1347, y=w1336) -> (x >= y?=w1346:bool)
                  n1197 = Concatenate Strings(w1339, w1337) -> (w1338:string)
                }
                "String 10" <- w1332
                n1198 = local write "Rd"(FALSE ("Boolean 7")) -> ()
              }
            }
          }
          frame #1 {
            w1359 = "_resized.jpg" ("command line")
            (unwired) ".jpg -resize 320x240 " ("string")
            (unwired) "Choose an Image File" ("prompt")
            # "-resize 1798x425"
            n1199 = local read "Image Path"() -> (w1353:path)
            n1200 = Strip Path(path=w1353) -> (stripped path=w1348:path, name=w1349:string)
            n1201 = Match Pattern(string=w1349, regular expression=".jpg") -> (before substring=→"before substring 2":string, after substring=→"after substring":string)  [unwired: 1 in, 2 out]
            n1202 = Match Pattern(string=w1349, regular expression="\\") -> (before substring=w1355:string)  [unwired: 1 in, 3 out]
            n1203 = Match Pattern(string=w1355, regular expression=".jpg") -> (before substring=w1354:string)  [unwired: 1 in, 3 out]
            n1204 = Concatenate Strings("cmd /c convert " ("string"), w1354, ".jpg -resize 320x240  " ("command line"), w1354, w1359) -> (w1362:string)
            n1205 = call <vilib>:"System Exec.vi"("run minimized? (F)"=TRUE, "wait until completion? (T)"=TRUE, "working directory"=w1348, "command line"=w1362) -> ("error out"=w1361:errorcluster)  [unwired: 4 in, 3 out]
            "error out 2" <- w1361
            n1206 = Concatenate Strings(w1354, w1359) -> (w1358:string)
          }
          frame #2 {
            n1207 = Wait (ms)(milliseconds to wait=u32 2000 ("millisecond timer value")) -> (millisecond timer value=w1367:u32)
          }
          frame #3 {
            n1208 = case shown="No Error" w1372 {
              tunnel: w1373 -> [w1376 _]
              tunnel: w1371 -> [w1374 _]
              frame No Error {
                (unwired) ".jpg" ("string")
                n1209 = Path To String(path=w1376) -> (string=w1380:string)
                n1210 = Concatenate Strings(w1380, "\\" ("string"), w1374) -> (w1379:string)
                n1211 = String To Path(string=w1379) -> (path=w1378:path)
                n1212 = call <vilib>:"Read JPEG File.vi"("path to JPEG file"=w1378) -> ("image data"=w1382:T16)  [unwired: 8 in, 2 out]
                "image data" <- w1382
                n1213 = local write "Print 3"(FALSE ("Print 2")) -> ()
                n1214 = call <vilib>:"Draw Flattened Pixmap.vi"("image data"=w1382) -> ("new picture"=→"new picture":picture)  [unwired: 8 in]
              }
              frame Error {
              }
            }
          }
        }
      }
    }
    n1215 = Wait (ms)(milliseconds to wait=u32 20 ("millisecond timer value")) -> ()  [unwired: 1 out]
    n1216 = local read "Quit"() -> (w1315:bool)
  }
  n1217 = while {
    tunnel: w38 -> [_]
    tunnel: w24 -> [_]
    stop <- w1412 stop-if-true
    # "New Adv Logics"
    n1218 = local read "Main Tab"() -> (w1393:T2)
    n1219 = local read "Main Tab"() -> (w1410:T2)
    n1220 = local read "Sign In"() -> (w1409:bool)
    n1221 = case shown="\"Adv Scar\"" w1393 {
      frame "HOME", Default {
        n1222 = local read "LIVE FEED MIN TEMP"() -> (w1545:bool)
        n1223 = local write "LIVE FEED MAX TEMP"(TRUE ("LIVE FEED MAX TEMP")) -> ()
        n1224 = local read "CAMERA ROI MIN TEMP"() -> (w1543:bool)
        n1225 = case shown="True" w1545 {
          selector: w1545 -> [_ w1552]
          frame False {
          }
          frame True {
            n1226 = Not(x=w1552) -> (.not. x?=w1551:bool)
            n1227 = local write "LIVE FEED MIN TEMP"(w1551) -> ()
            n1228 = call "CAMERA LIVE FEED FGV.vi"("Enum - Menu"=CAMERA_LIVE_FEED_ENUM."CAMERA MINIMIZE") -> ()  [unwired: 9 in, 2 out]
          }
        }
        n1229 = case shown="True" w1543 {
          selector: w1543 -> [_ w1549]
          frame False {
          }
          frame True {
            n1230 = Not(x=w1549) -> (.not. x?=w1548:bool)
            n1231 = local write "CAMERA ROI MIN TEMP"(w1548) -> ()
            n1232 = call "IMAGE ANALYSIS.vi"("Enum"=POST_ANALYSIS_ENUM."MINIMIZE UI") -> ()  [unwired: 9 in, 2 out]
          }
        }
        n1233 = local write "CAMERA ROI MAX TEMP"(TRUE ("CAMERA ROI MAX TEMP")) -> ()
      }
      frame "Test Setup" {
        n1234 = local read "LIVE FEED MIN TEMP"() -> (w1555:bool)
        n1235 = local read "CAMERA ROI MIN TEMP"() -> (w1553:bool)
        n1236 = local write "LIVE FEED MAX TEMP"(TRUE ("LIVE FEED MAX TEMP")) -> ()
        n1237 = case shown="True" w1555 {
          selector: w1555 -> [_ w1562]
          frame False {
          }
          frame True {
            n1238 = Not(x=w1562) -> (.not. x?=w1561:bool)
            n1239 = local write "LIVE FEED MIN TEMP"(w1561) -> ()
            n1240 = call "CAMERA LIVE FEED FGV.vi"("Enum - Menu"=CAMERA_LIVE_FEED_ENUM."CAMERA MINIMIZE") -> ()  [unwired: 9 in, 2 out]
          }
        }
        n1241 = case shown="True" w1553 {
          selector: w1553 -> [_ w1559]
          frame False {
          }
          frame True {
            n1242 = Not(x=w1559) -> (.not. x?=w1558:bool)
            n1243 = local write "CAMERA ROI MIN TEMP"(w1558) -> ()
            n1244 = call "IMAGE ANALYSIS.vi"("Enum"=POST_ANALYSIS_ENUM."MINIMIZE UI") -> ()  [unwired: 9 in, 2 out]
          }
        }
        n1245 = local write "CAMERA ROI MAX TEMP"(TRUE ("CAMERA ROI MAX TEMP")) -> ()
      }
      frame "Acquire" {
        n1246 = local read "LIVE FEED MIN TEMP"() -> (w1565:bool)
        n1247 = local write "LIVE FEED MAX TEMP"(TRUE ("LIVE FEED MAX TEMP")) -> ()
        n1248 = local read "CAMERA ROI MIN TEMP"() -> (w1563:bool)
        n1249 = case shown="True" w1565 {
          selector: w1565 -> [_ w1572]
          frame False {
          }
          frame True {
            n1250 = Not(x=w1572) -> (.not. x?=w1571:bool)
            n1251 = local write "LIVE FEED MIN TEMP"(w1571) -> ()
            n1252 = call "CAMERA LIVE FEED FGV.vi"("Enum - Menu"=CAMERA_LIVE_FEED_ENUM."CAMERA MINIMIZE") -> ()  [unwired: 9 in, 2 out]
          }
        }
        n1253 = case shown="True" w1563 {
          selector: w1563 -> [_ w1569]
          frame False {
          }
          frame True {
            n1254 = Not(x=w1569) -> (.not. x?=w1568:bool)
            n1255 = local write "CAMERA ROI MIN TEMP"(w1568) -> ()
            n1256 = call "IMAGE ANALYSIS.vi"("Enum"=POST_ANALYSIS_ENUM."MINIMIZE UI") -> ()  [unwired: 9 in, 2 out]
          }
        }
        n1257 = local write "CAMERA ROI MAX TEMP"(TRUE ("CAMERA ROI MAX TEMP")) -> ()
      }
      frame "Adv Scar" {
        n1258 = local read "CAMERA ROI MIN TEMP"() -> (w1573:bool)
        n1259 = case shown="True" "LIVE FEED MAX TEMP" {
          selector: "LIVE FEED MAX TEMP" -> [_ w1594]
          frame False {
          }
          frame True {
            n1260 = Not(x=w1594) -> (.not. x?=w1593:bool)
            n1261 = local write "LIVE FEED MAX TEMP"(w1593) -> ()
            n1262 = call "CAMERA LIVE FEED FGV.vi"("Enum - Menu"=CAMERA_LIVE_FEED_ENUM."CAMERA RESTORE") -> ("error out"=w1584:errorcluster)  [unwired: 9 in, 1 out]
            n1263 = Type Cast(type=30, x=0) -> (*(type *) &x=w1588:i32)
            n1264 = Add(x=w1588, y=48) -> (x+y=w1589:i32)
            n1265 = call "CAMERA LIVE FEED FGV.vi"("Enum - Menu"=CAMERA_LIVE_FEED_ENUM."CAMERA MODE SET", "error in (no error)"=w1584, "CAMERA MODE"=w1589) -> ("error out"=w1581:errorcluster)  [unwired: 7 in, 1 out]
            n1266 = call "CAMERA LIVE FEED FGV.vi"("Enum - Menu"=CAMERA_LIVE_FEED_ENUM."CAMERA GRAY", "error in (no error)"=w1581) -> ("error out"=w1580:errorcluster)  [unwired: 8 in, 1 out]
            n1267 = call "LIST FILE NAMES.vi"("error in (no error)"=w1580) -> ("error out"=w1590:errorcluster, "filenames"=w1591:string[])  [unwired: 9 in]
            n1268 = property on="FILE 3" class="CmbBox"(error in=w1590, "Strings[]"=w1591) -> ()  [unwired: 1 in, 2 out]
          }
        }
        n1269 = case shown="True" w1573 {
          selector: w1573 -> [_ w1579]
          frame False {
          }
          frame True {
            n1270 = Not(x=w1579) -> (.not. x?=w1578:bool)
            n1271 = local write "CAMERA ROI MIN TEMP"(w1578) -> ()
            n1272 = call "IMAGE ANALYSIS.vi"("Enum"=POST_ANALYSIS_ENUM."MINIMIZE UI") -> ()  [unwired: 9 in, 2 out]
          }
        }
        n1273 = local write "CAMERA ROI MAX TEMP"(TRUE ("CAMERA ROI MAX TEMP")) -> ()
        "LIVE FEED MIN TEMP" <- TRUE ("LIVE FEED MIN TEMP")
      }
      frame "Adv Scar Report" {
        n1274 = local read "CAMERA ROI MAX TEMP"() -> (w1595:bool)
        n1275 = local read "LIVE FEED MIN TEMP"() -> (w1597:bool)
        n1276 = local write "LIVE FEED MAX TEMP"(TRUE ("LIVE FEED MAX TEMP")) -> ()
        n1277 = case shown="True" w1597 {
          selector: w1597 -> [_ w1606]
          frame False {
          }
          frame True {
            n1278 = Not(x=w1606) -> (.not. x?=w1605:bool)
            n1279 = local write "LIVE FEED MIN TEMP"(w1605) -> ()
            n1280 = call "CAMERA LIVE FEED FGV.vi"("Enum - Menu"=CAMERA_LIVE_FEED_ENUM."CAMERA MINIMIZE") -> ()  [unwired: 9 in, 2 out]
          }
        }
        n1281 = case shown="True" w1595 {
          selector: w1595 -> [_ w1603]
          frame False {
          }
          frame True {
            n1282 = Not(x=w1603) -> (.not. x?=w1601:bool)
            n1283 = local write "CAMERA ROI MAX TEMP"(w1601) -> ()
            n1284 = call "IMAGE ANALYSIS.vi"("Enum"=POST_ANALYSIS_ENUM."SHOW UI") -> ("error out"=w1600:errorcluster)  [unwired: 9 in, 1 out]
            n1285 = call "LIST FILE NAMES.vi"("error in (no error)"=w1600) -> ("filenames"=w1599:string[])  [unwired: 9 in, 1 out]
            n1286 = property on="Test File List :" class="CmbBox"("Strings[]"=w1599) -> ()  [unwired: 2 in, 2 out]
          }
        }
        n1287 = local write "CAMERA ROI MIN TEMP"(TRUE ("CAMERA ROI MIN TEMP")) -> ()
      }
      frame "Compare Files" {
        n1288 = local read "LIVE FEED MIN TEMP"() -> (w1609:bool)
        n1289 = local write "LIVE FEED MAX TEMP"(TRUE ("LIVE FEED MAX TEMP")) -> ()
        n1290 = local read "CAMERA ROI MIN TEMP"() -> (w1607:bool)
        n1291 = case shown="True" w1609 {
          selector: w1609 -> [_ w1616]
          frame False {
          }
          frame True {
            n1292 = Not(x=w1616) -> (.not. x?=w1615:bool)
            n1293 = local write "LIVE FEED MIN TEMP"(w1615) -> ()
            n1294 = call "CAMERA LIVE FEED FGV.vi"("Enum - Menu"=CAMERA_LIVE_FEED_ENUM."CAMERA MINIMIZE") -> ()  [unwired: 9 in, 2 out]
          }
        }
        n1295 = case shown="True" w1607 {
          selector: w1607 -> [_ w1613]
          frame False {
          }
          frame True {
            n1296 = Not(x=w1613) -> (.not. x?=w1612:bool)
            n1297 = local write "CAMERA ROI MIN TEMP"(w1612) -> ()
            n1298 = call "IMAGE ANALYSIS.vi"("Enum"=POST_ANALYSIS_ENUM."MINIMIZE UI") -> ()  [unwired: 9 in, 2 out]
          }
        }
        n1299 = local write "CAMERA ROI MAX TEMP"(TRUE ("CAMERA ROI MAX TEMP")) -> ()
      }
      frame "About" {
        n1300 = local read "LIVE FEED MIN TEMP"() -> (w1619:bool)
        n1301 = local write "LIVE FEED MAX TEMP"(TRUE ("LIVE FEED MAX TEMP")) -> ()
        n1302 = local read "CAMERA ROI MIN TEMP"() -> (w1618:bool)
        n1303 = case shown="True" w1619 {
          selector: w1619 -> [_ w1626]
          frame False {
          }
          frame True {
            n1304 = Not(x=w1626) -> (.not. x?=w1625:bool)
            n1305 = local write "LIVE FEED MIN TEMP"(w1625) -> ()
            n1306 = call "CAMERA LIVE FEED FGV.vi"("Enum - Menu"=CAMERA_LIVE_FEED_ENUM."CAMERA MINIMIZE") -> ()  [unwired: 9 in, 2 out]
          }
        }
        n1307 = case shown="True" w1618 {
          selector: w1618 -> [_ w1623]
          frame False {
          }
          frame True {